vi "Trajectory Builder.vi"() -> ()   [LabVIEW 2025] (continued)
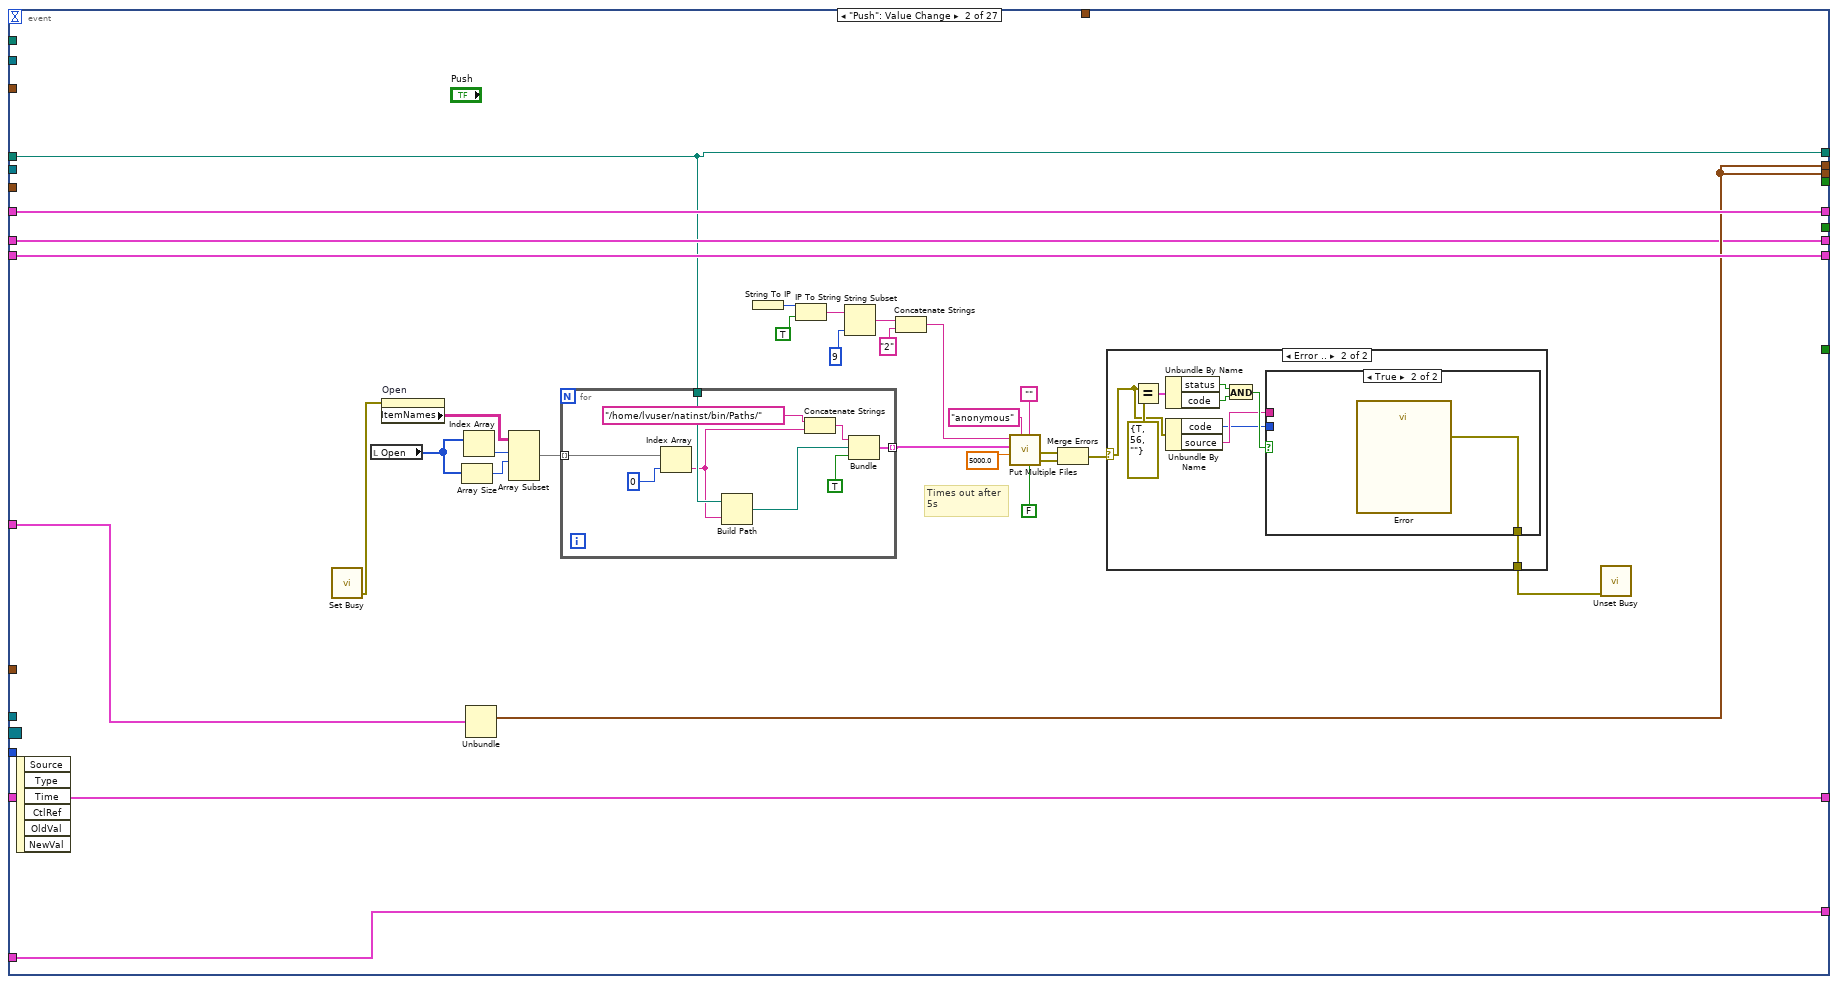
[diagram p4: hidden frame]
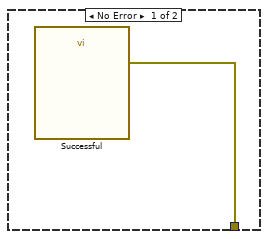
[diagram p5: hidden frame]
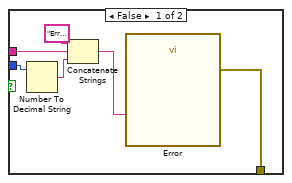
[diagram p6: hidden frame]
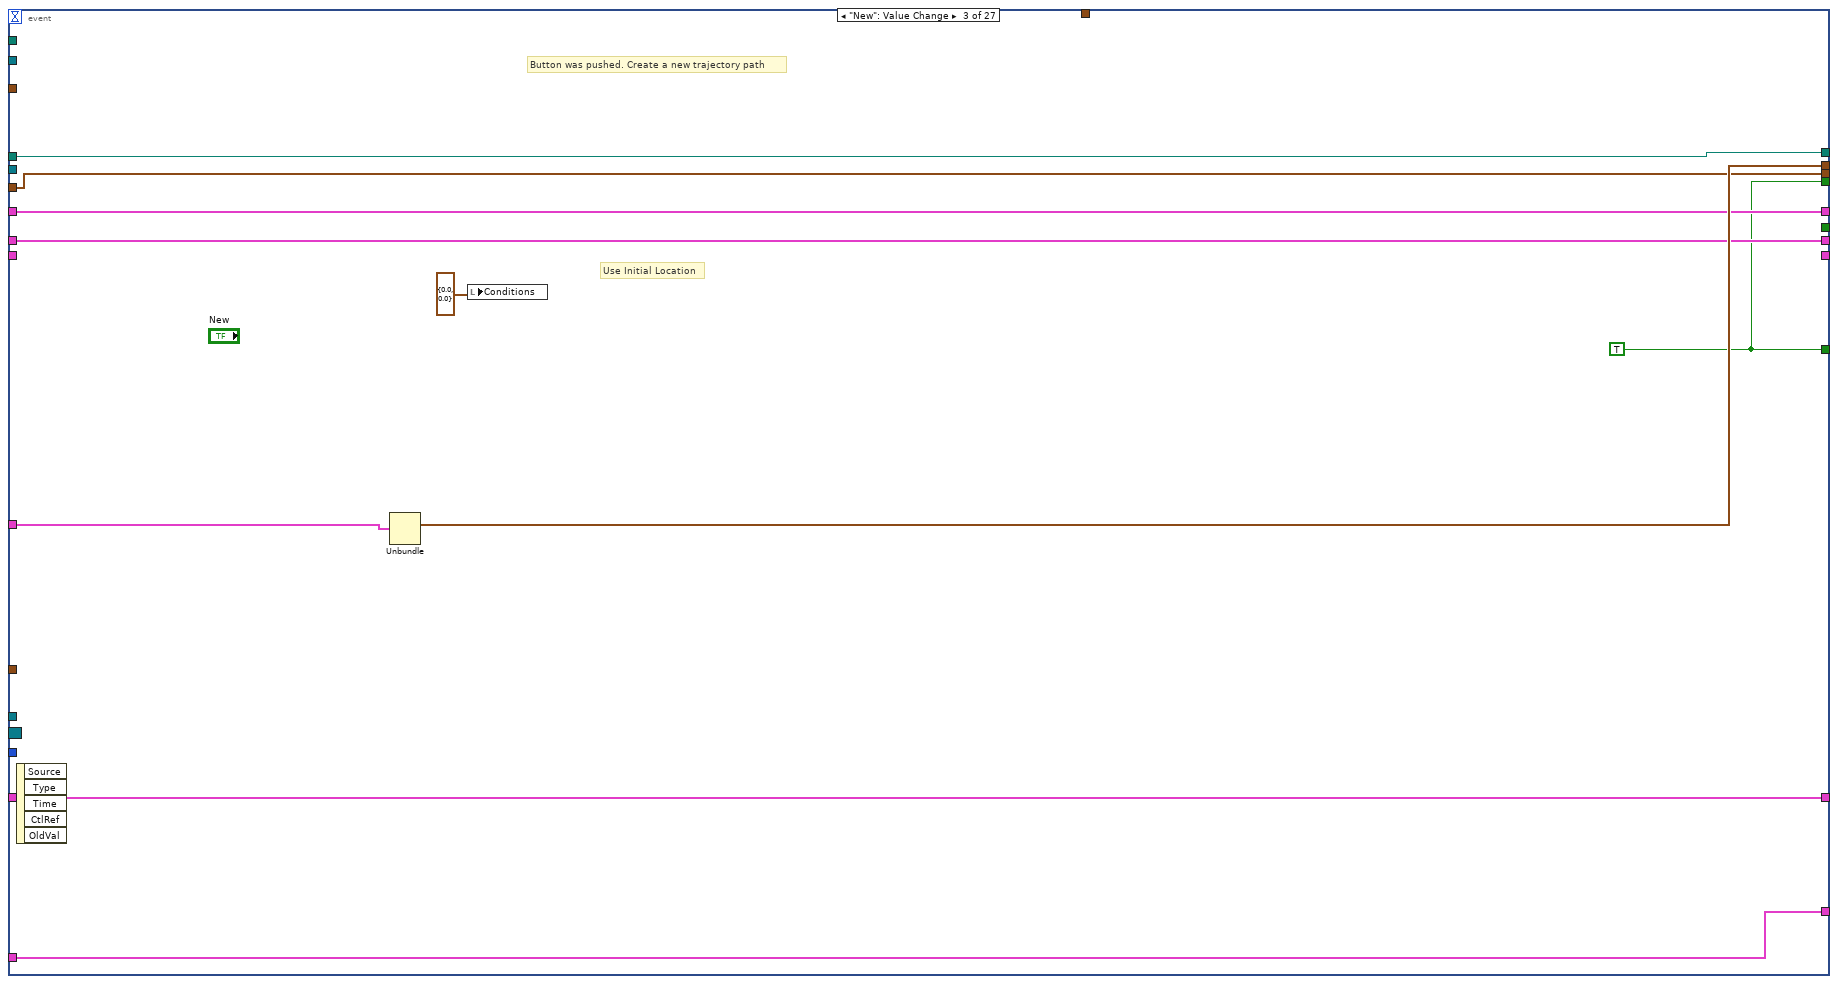
[diagram p7: hidden frame]
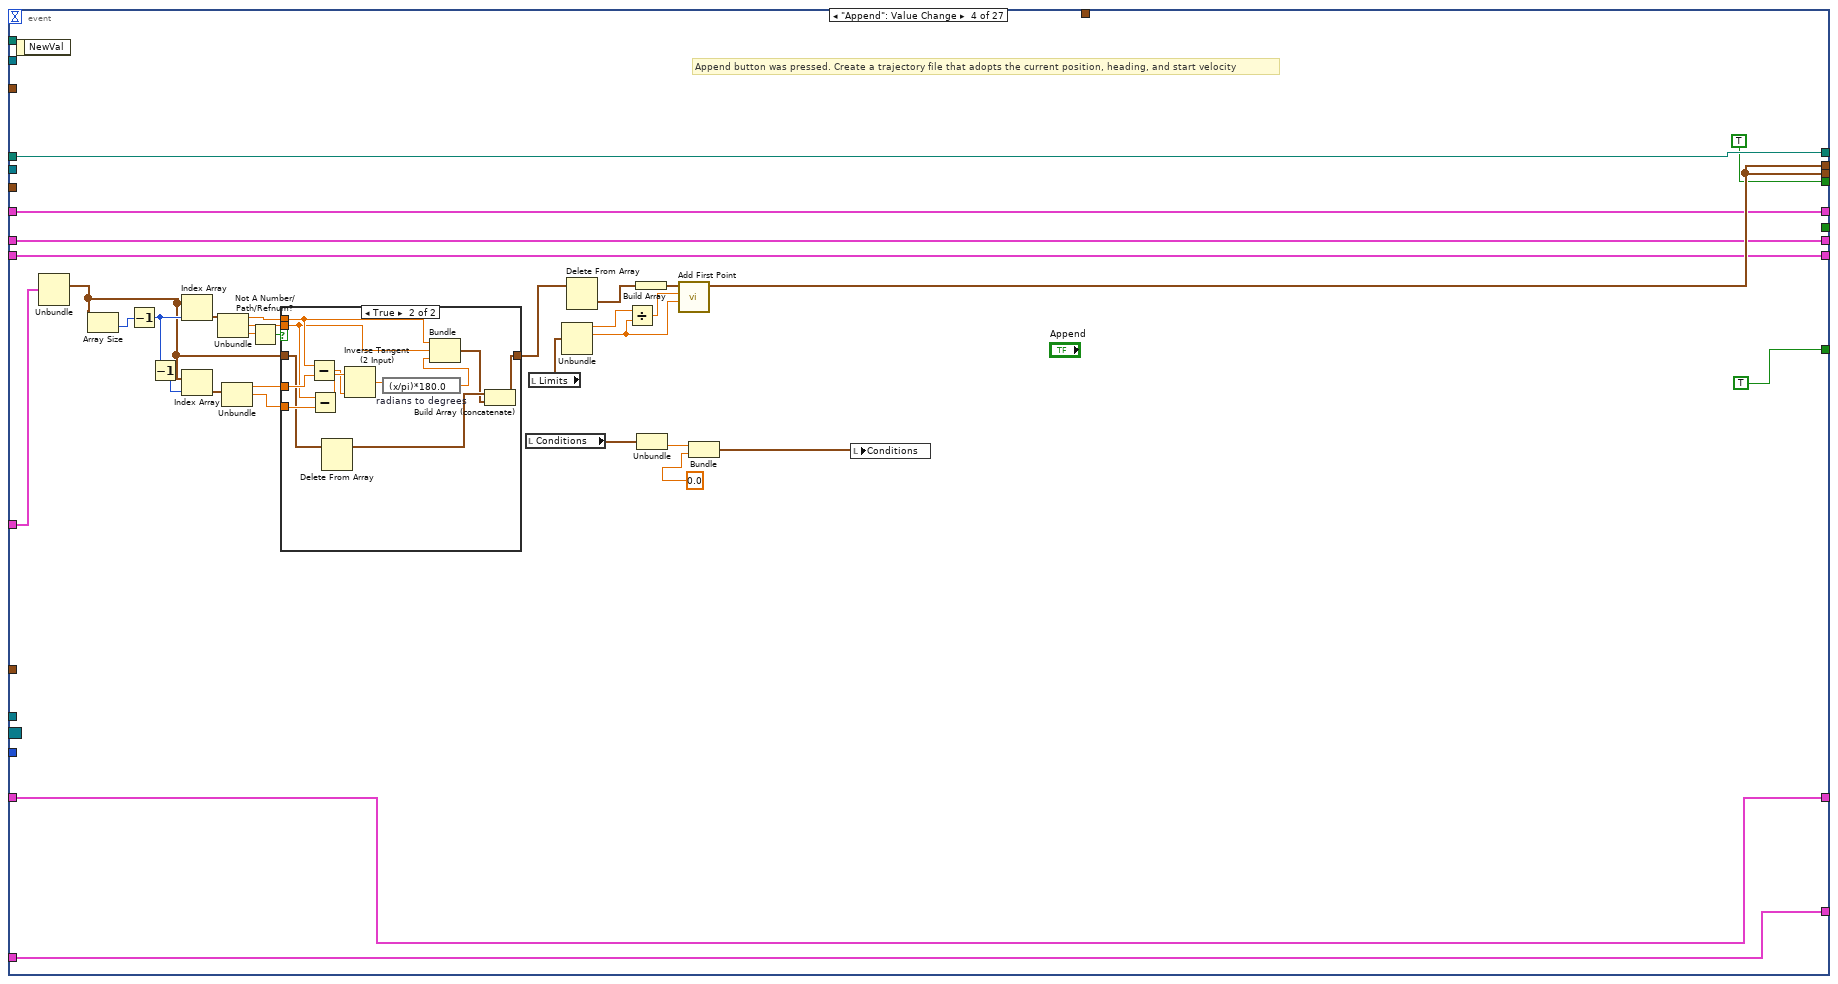
[diagram p8: hidden frame]
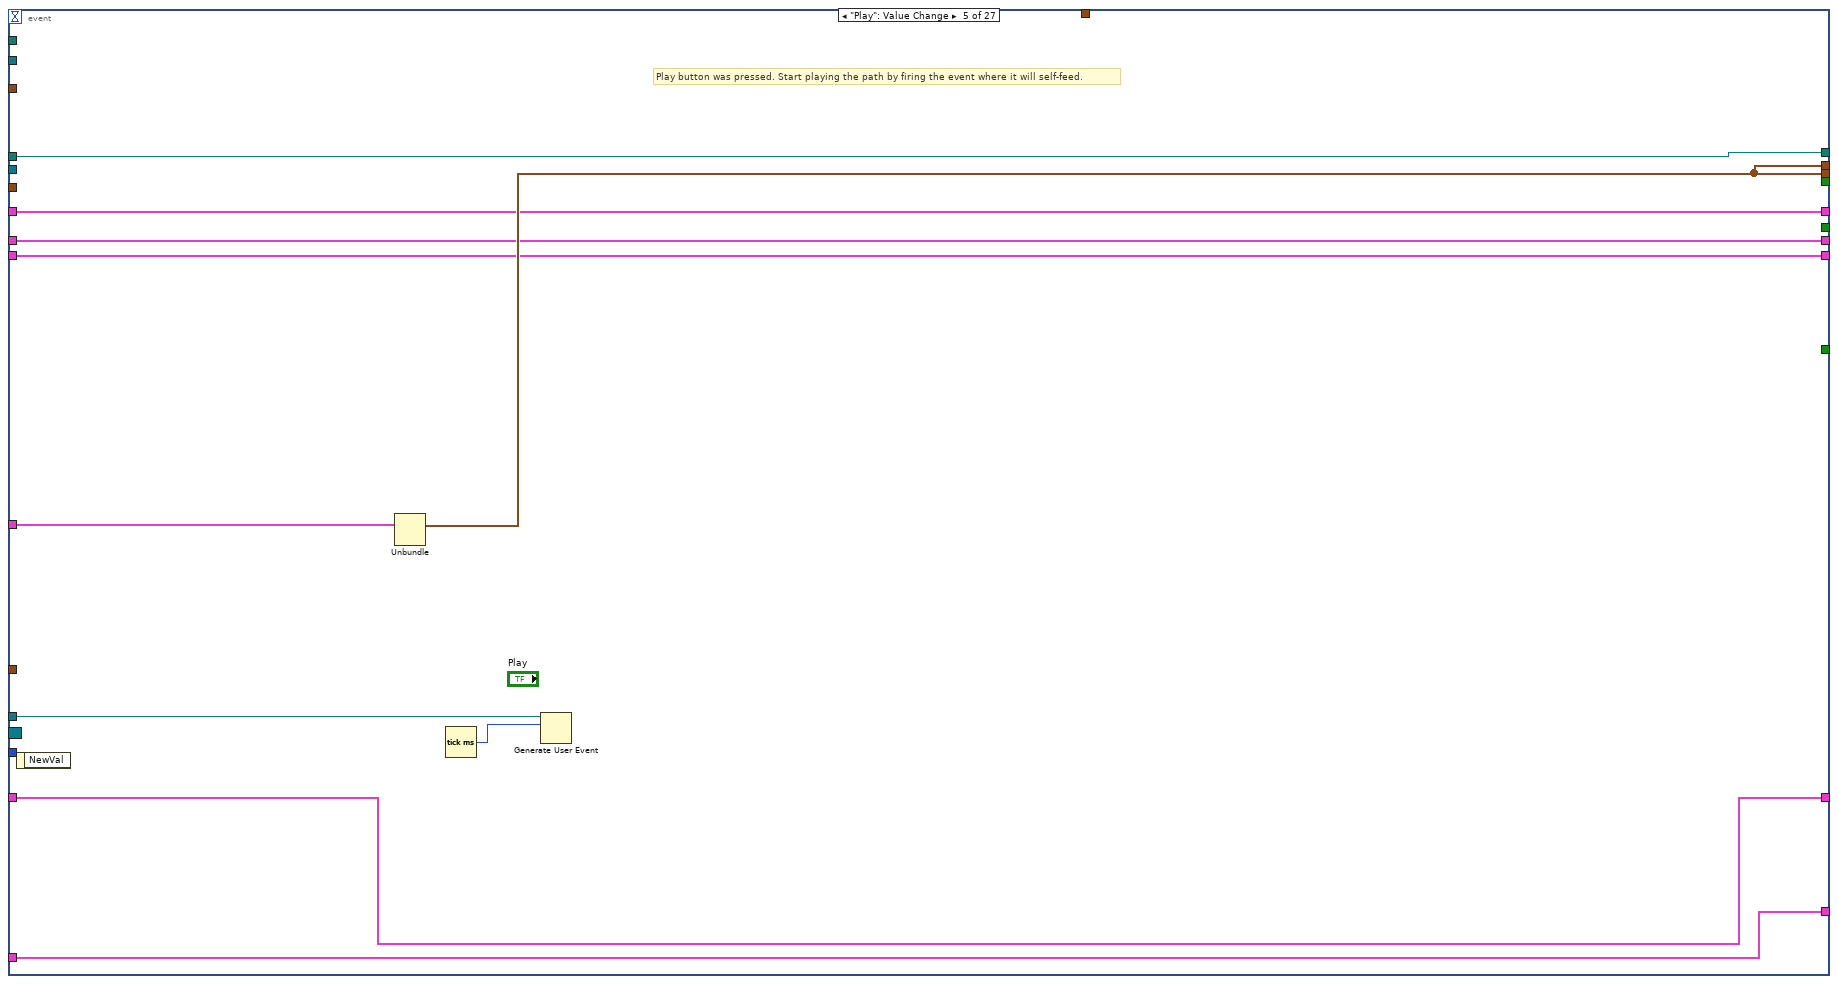
[diagram p10: hidden frame]
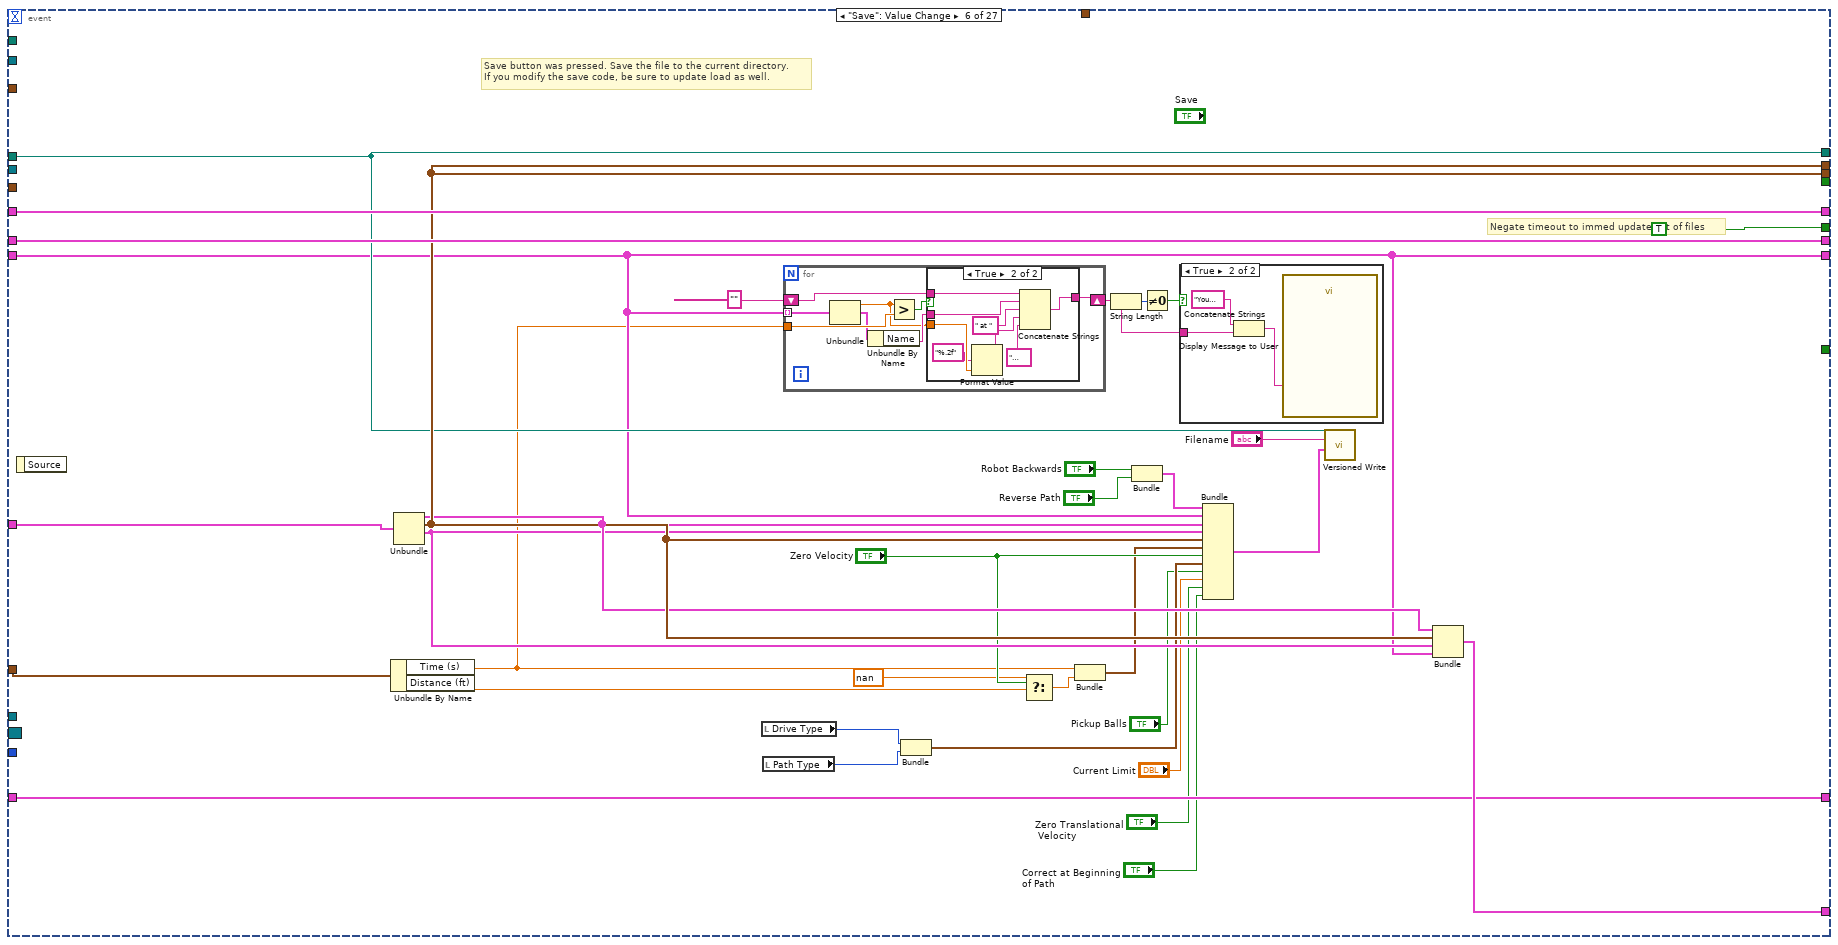
[diagram p11: hidden frame]
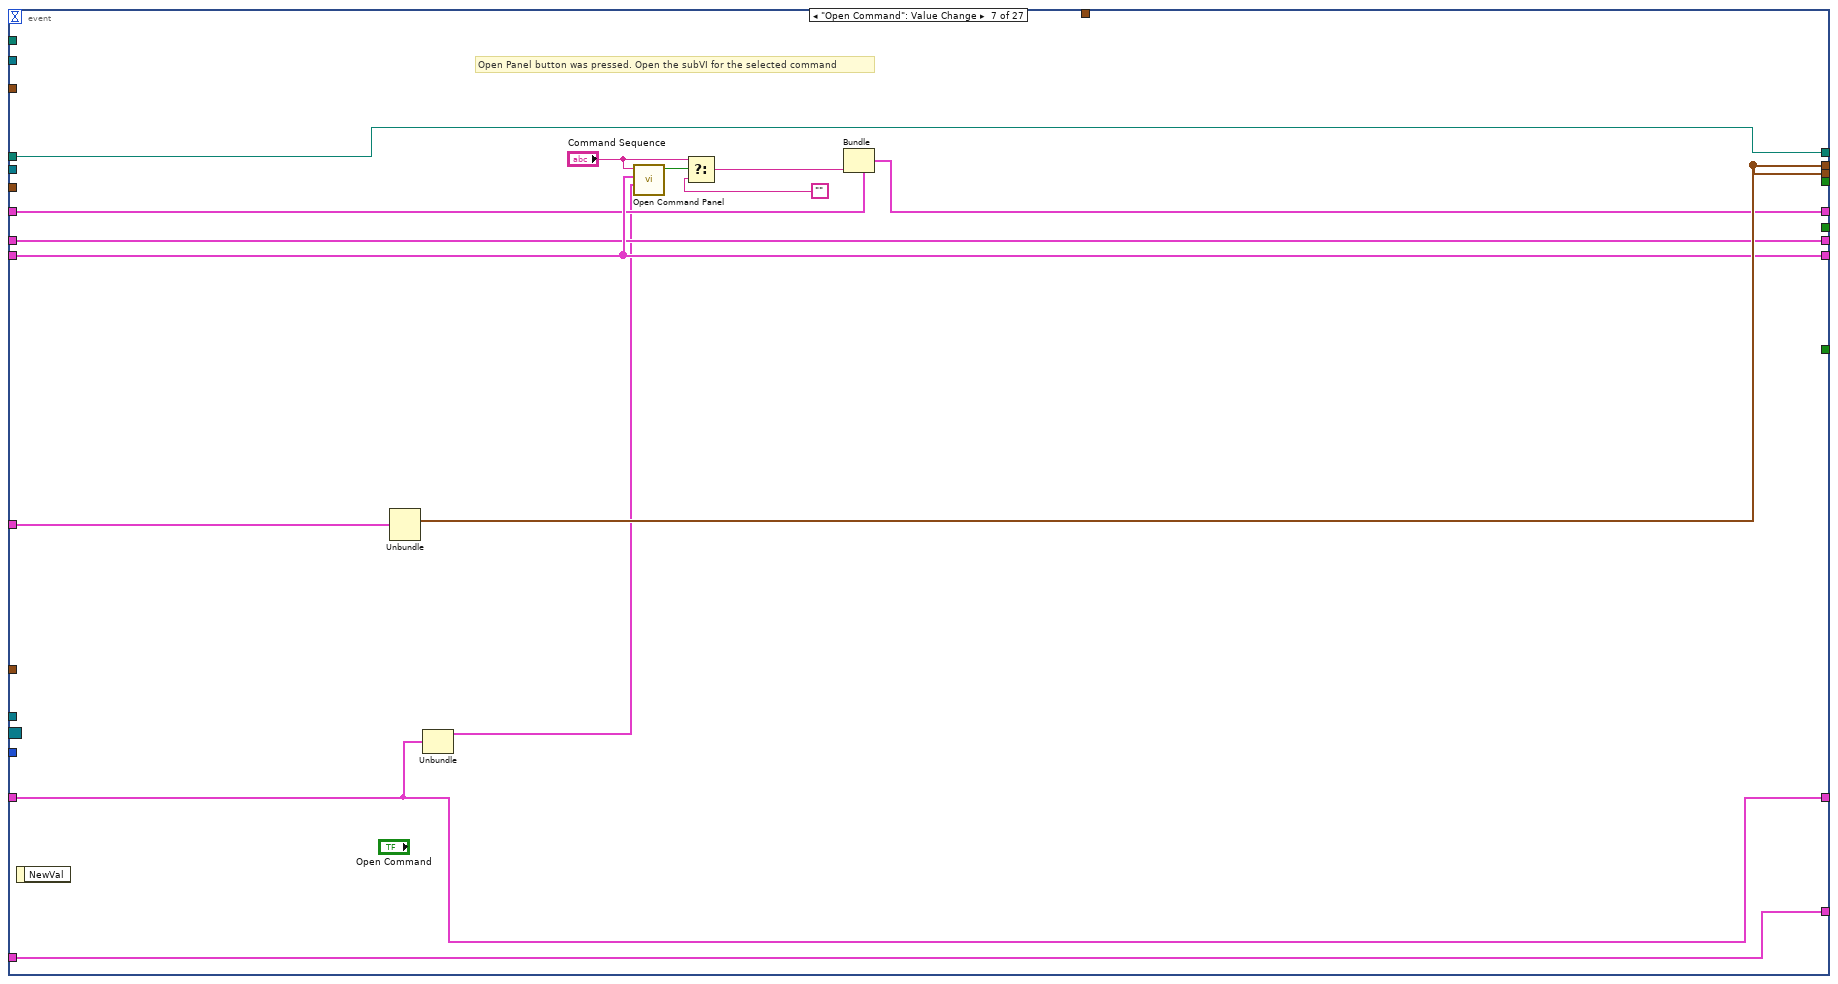
[diagram p14: hidden frame]
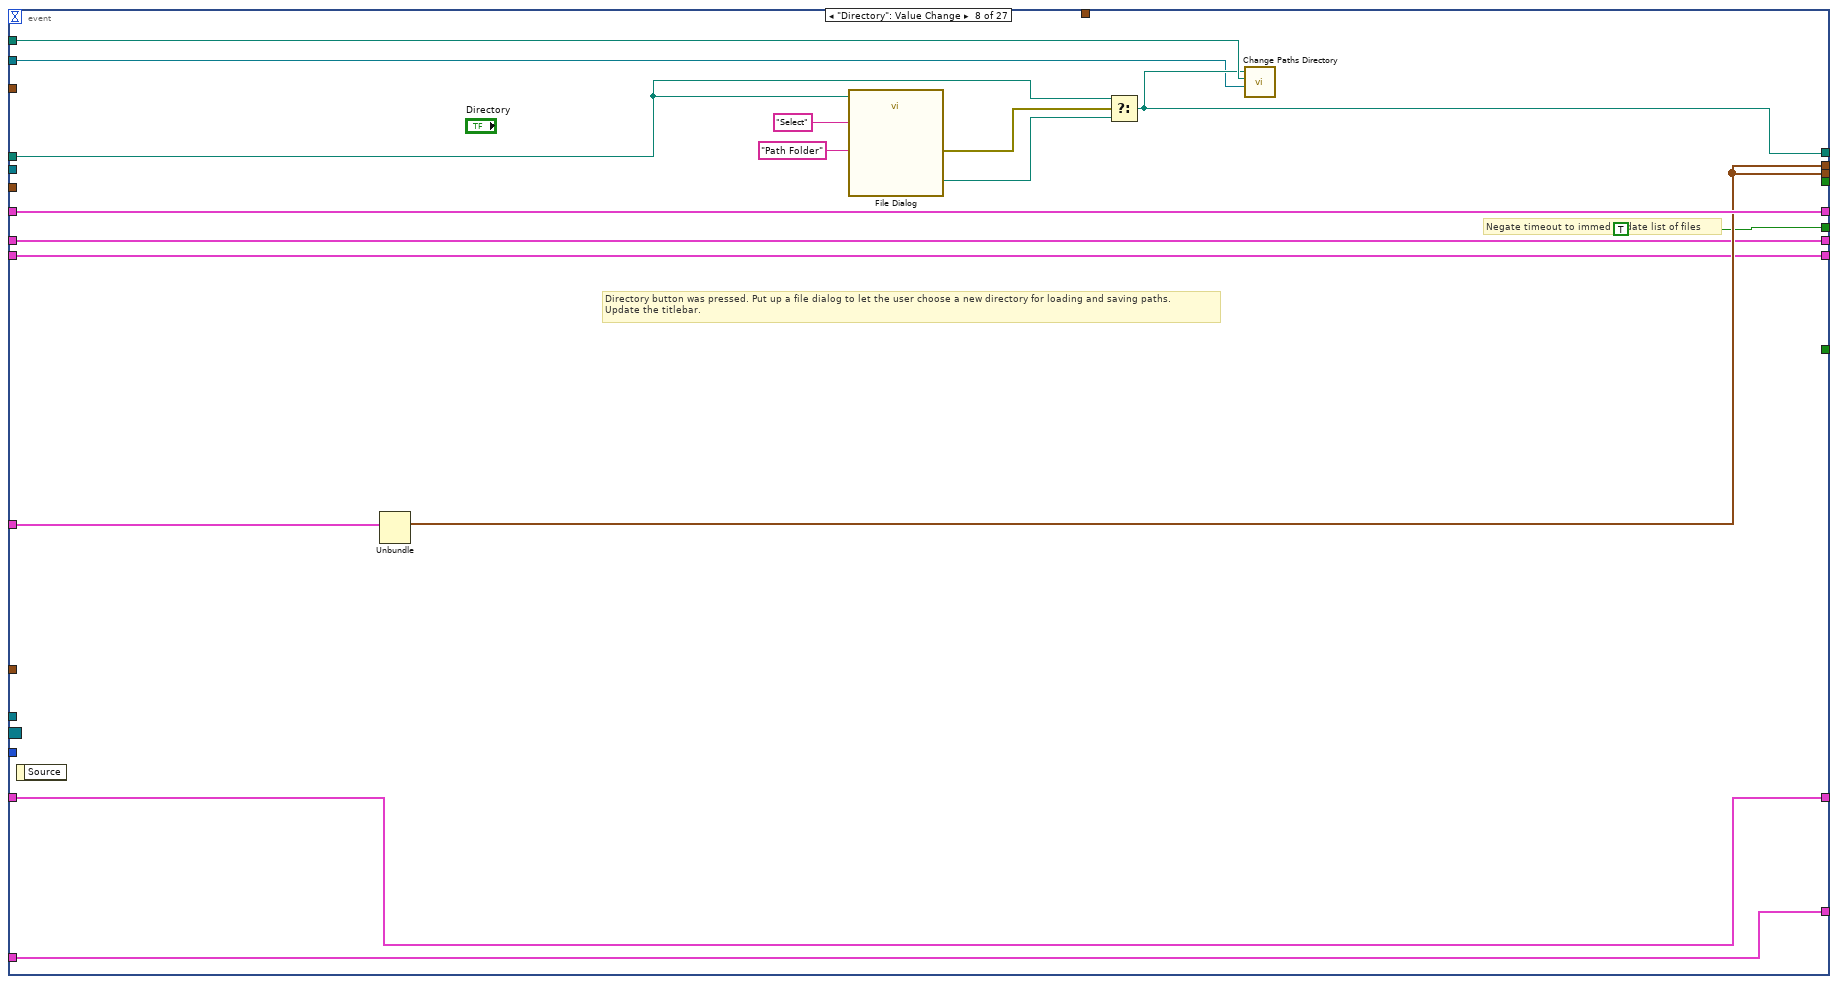
[diagram p15: hidden frame]
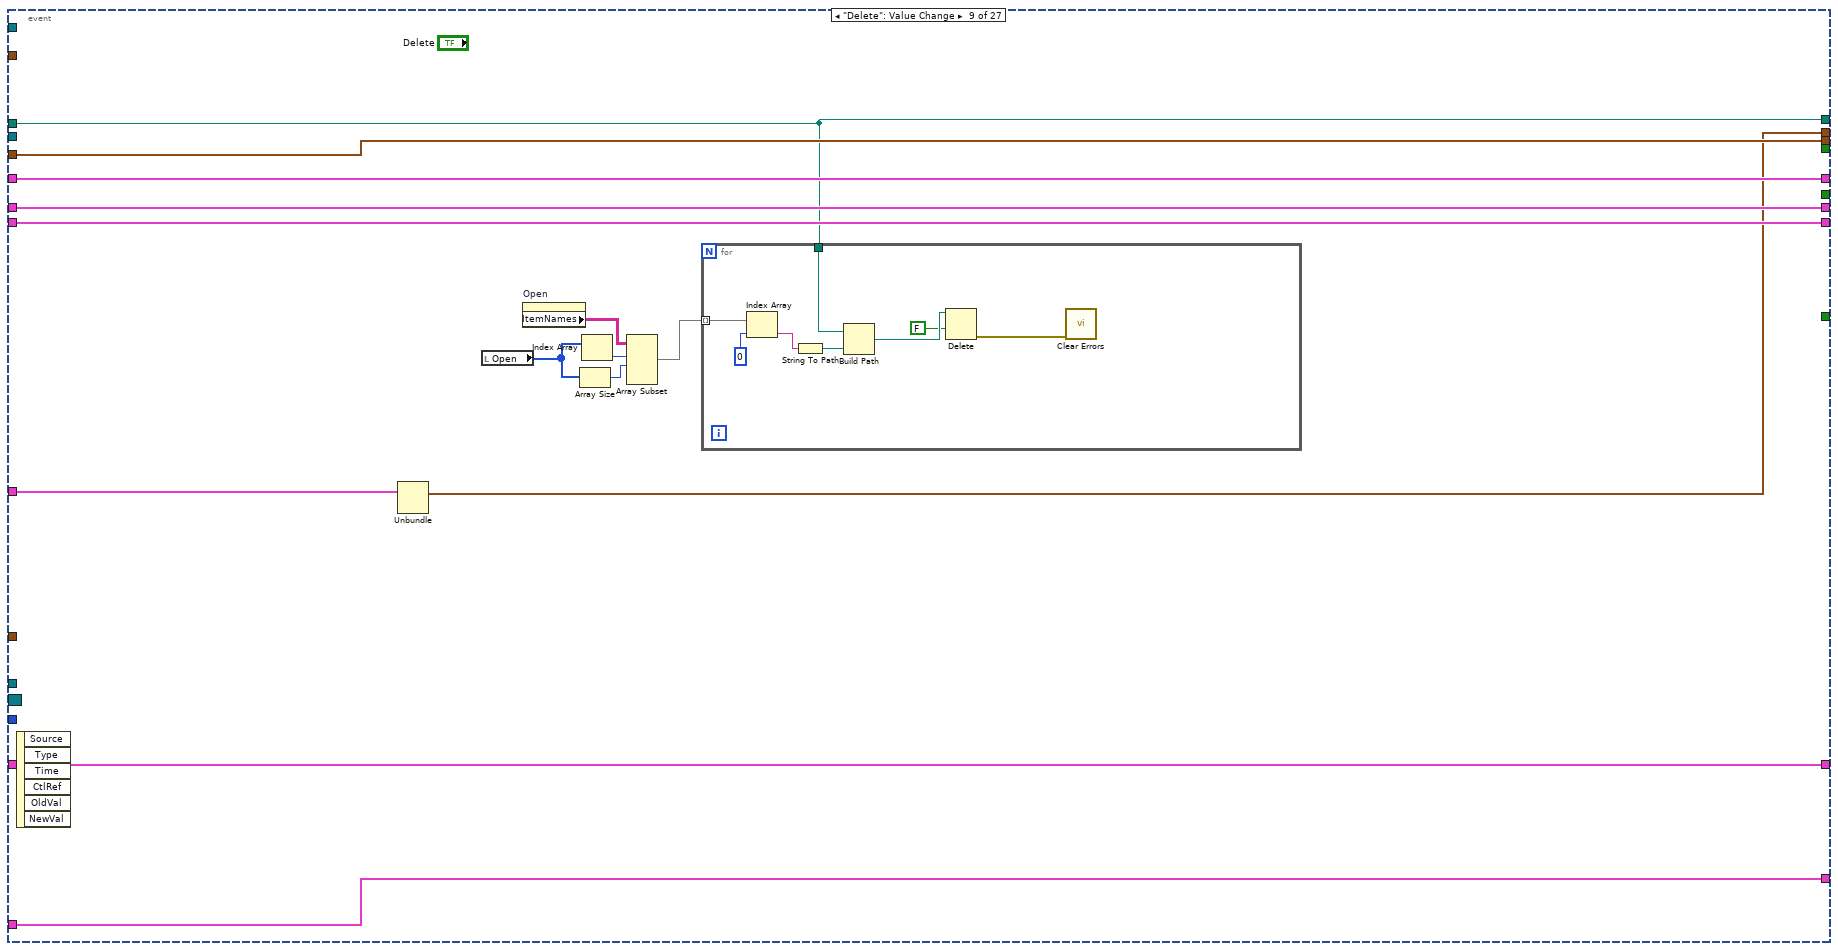
[diagram p16: hidden frame]
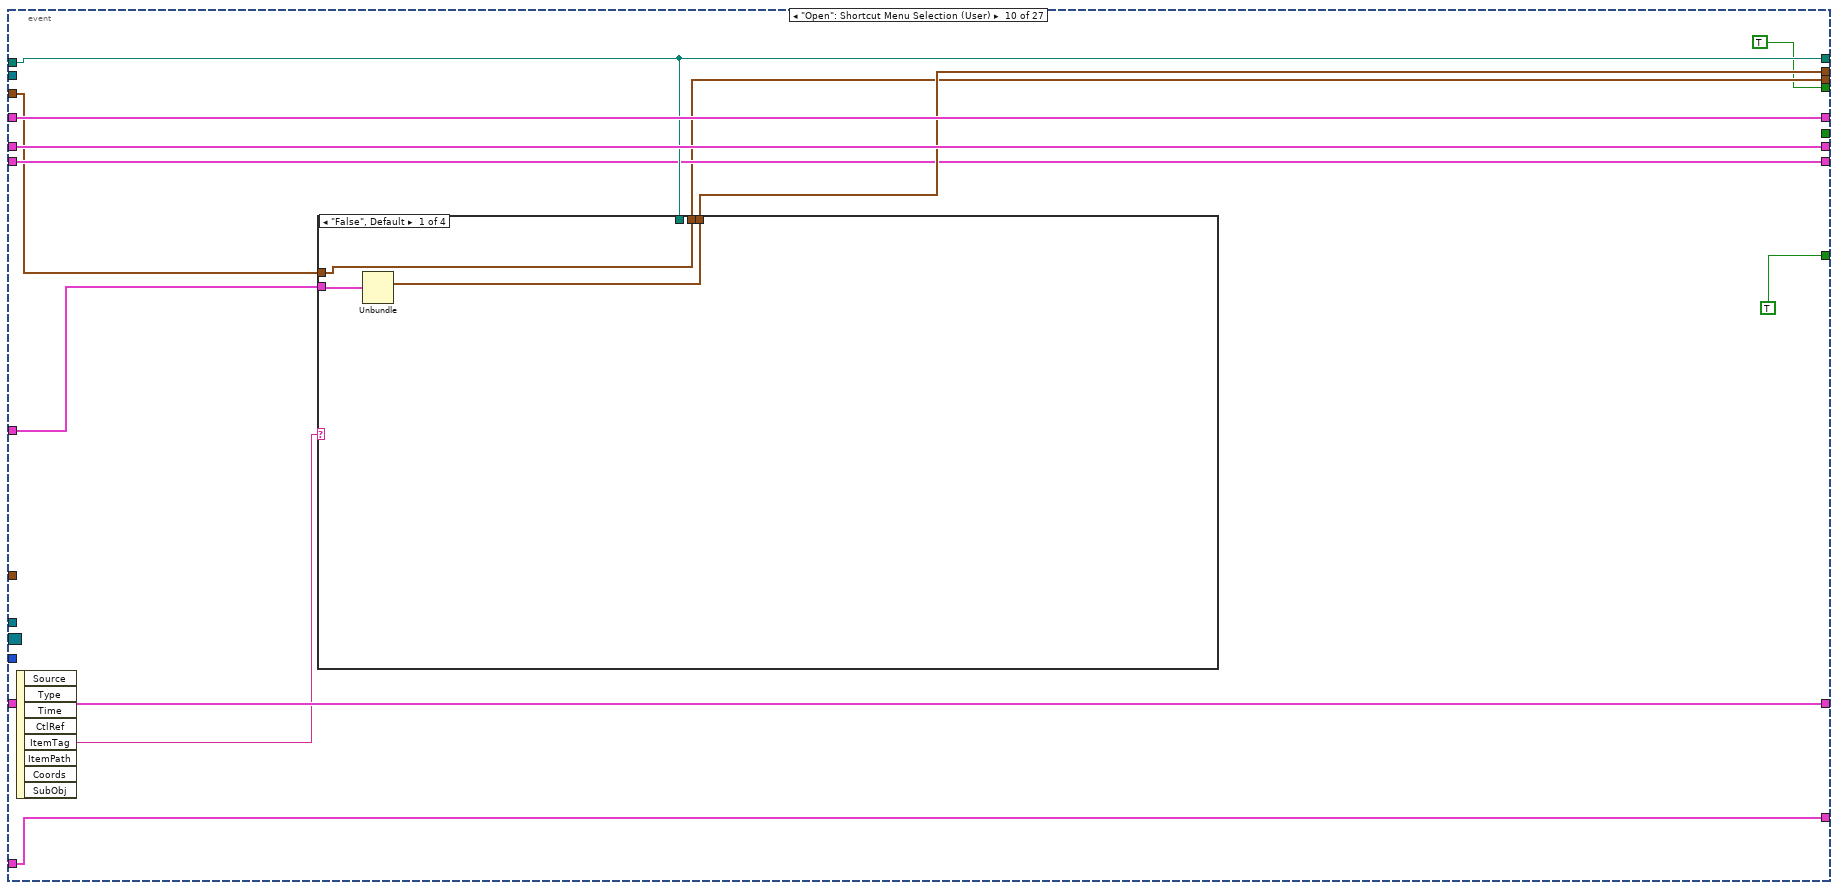
[diagram p17: hidden frame]
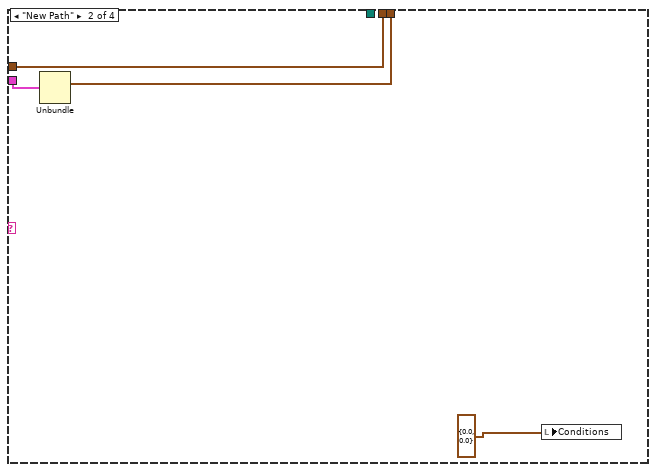
[diagram p18: hidden frame]
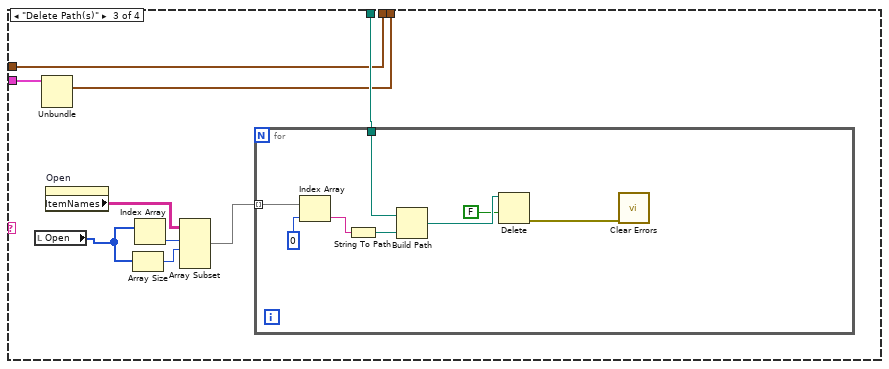
[diagram p19: hidden frame]
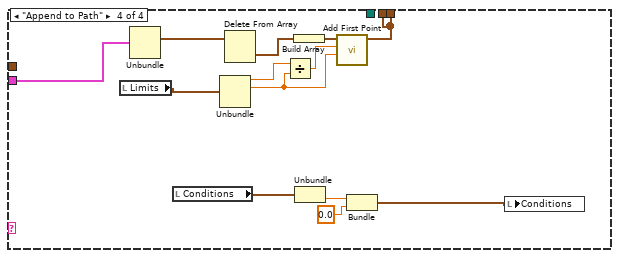
[diagram p20: hidden frame]
    n508 = flat-sequence {
      tunnel: ["Time (s)"] -> w113
      tunnel: ["Sample Period (s)"] -> w86
      tunnel: ["Limits"] -> w65
      tunnel: ["Conditions"] -> w51
      tunnel: [w128] -> w75
      tunnel: ["Overrides"] -> w50
      tunnel: w79 -> [w128]
      tunnel: w78 -> [w130]
      tunnel: ["Hide Path"] -> w69
      tunnel: ["Stoopid Overlap %"] -> w68
      tunnel: ["Angular Limits"] -> w49
      tunnel: [w122] -> w46
      frame #0 {
        n509 = control-ref of="Command Sequence"() -> (w131:refnum<vi>)
        n510 = global write "Global Settings.vi" "> 90?"("Allow Angles > 90") -> ()
        n511 = global write "Global Settings.vi" "Turn Angle Limit (deg)"("Turn Angle Limit (deg)") -> ()
        n512 = call "Format Tree.vi"("Update"=w130, "Commands"=w128, "Tree Refnum"=w131) -> ()  [unwired: 9 in]
        n513 = local read "Overrides"() -> (w122:T8)
      }
    }
    n514 = Unbundle(w65) -> ("Accel (fps^2)"=w64:dbl)  [unwired: 3 out]
    n515 = Divide(x=w113, y=w86) -> (x/y=w106:dbl)
    n516 = Bundle("Sample Period (s)"=w86, "Limits"=w65, "Conditions"=w51, "Overrides"=w50, "Angular Limits"=w49) -> (w66:T14)  [unwired: 1 in]
    n517 = call "Enforce Robot Rules.vi"("max V"=w71, "Drive Type"="Drive Type", "Overrides"=w46, "turn accel"=w64, "Disable"=w59, "New Points"=w108, "Original Points"=w107) -> ("Overrides Out"=w52:T8, "Points out"=w48:cluster{"x":dbl, "y":dbl, "th":dbl}[])  [unwired: 3 in]
    n518 = call "GenNewTraj.vi"("Drive Type"="Drive Type", "Turn Rate"="Turn Rate (Bezier)", "Stoopid Overlap %"=w68, "Path Type"="Path Type", "Parameters"=w66, "Points in"=w48) -> ("Time & Dist"=w58:cluster{"Time (s)":dbl, "Distance (ft)":dbl}, "Valid"=w87:bool, "Trajectory Data"=w95:T12, "Updated Waypoints"=w99:cluster{"x":dbl, "y":dbl, "th":dbl}[])  [unwired: 2 in]
    "Trajectory Data" <- w95
    n519 = local write "WayPoints"(w48) -> ()
    n520 = local write "Overrides"(w52) -> ()
    n521 = Unbundle(w58) -> ("Time (s)"=w56:dbl, "Distance (ft)"=→"Distance (ft)":dbl)
    "Duration (s)" <- w56
    n522 = Unbundle(w93) -> ("Hover Object"=w92:T17)  [unwired: 2 out]
    n523 = Bundle(cluster=T20 {"Trajectory Data"=[], "Updated Waypoints"=[], {"Sample Period (s)"=0.0, "Limits"={"Velocity (fps)"=0.0, "Accel (fps^2)"=0.0, "Jerk (fps^3)"=0.0, "StoopidFast (fps)"=0.0}, "Conditions"={"vInitial (fps)"=0.0, "vFinal (fps)"=0.0}, "Overrides"=[], "Angular Limits"={"Velocity (deg/s)"=6.0, "Accel (deg/s^2)"=15.0, "Jerk (deg/s^3)"=150.0}}, "Commands out"=[]} ("output cluster"), "Trajectory Data"=w95, "Updated Waypoints"=w99, w66, "Commands out"=w75) -> (w53:T20)
    n524 = property on="Time (s)" class="Slide (strict)"("Scale.Minimum"=0.0 ("Scale.Range:Minimum"), "Scale.Maximum"=w56) -> ()  [unwired: 2 in, 2 out]
    n525 = call "Draw Trajectory.vi"("Robot Index"=w106, "Hide Path"=w69, "new picture in"=picture data[5B] ("new picture"), "Trajectory Data"=w95, "Picture in"=w116) -> ("Path Points"=w100:cluster{"x":dbl, "y":dbl}[], "Output Point"=w112:T39, "new picture"=w114:picture)  [unwired: 4 in]
    n526 = call "Draw Shapes.vi"("Path Points"=w100, "Sample Period (s)"=w86, "Output Point"=w112, "Commands"=w75, "Results"=w92, "new picture in"=w114, "Points"=w99, "Picture in"=w116) -> ("new picture out"=→"Picture":picture)  [unwired: 3 in]
    n527 = call "Update Annotations.vi"("Sample Period"=w86, "Commands"=w75, "Trajectory Data"=w95, "Robot Pt Index"=w106) -> ("Redraw"=w77:bool, "Velocity Trace"=w76:dbl[], "Annotation Data"=w105:T40)  [unwired: 5 in]
    n528 = case shown="True" w77 {
      tunnel: w105 -> [_ w1156]
      tunnel: w76 -> [_ w1155]
      frame False {
      }
      frame True {
        n529 = property on="fps" class="WFGraph (strict)"("AnntList"=w1156) -> ()  [unwired: 2 in, 2 out]
        "fps" <- w1155
      }
    }
    n530 = disable-structure shown="Disabled" {
      disable-tunnel: w87 -> [w119 _]
      frame Disabled {
        n531 = Select(t=cluster{u32, u32}[] [{14869218, 14869218}] ("Colors [4]"), s=w119, f=cluster{u32, u32}[] [{6094681, 6094681}] ("Colors [4]")) -> ()  [unwired: 1 out]
      }
      frame Enabled {
      }
    }
    n532 = control-ref of="Save"() -> (w62:refnum<vi>)
    n533 = Select(t=0, s=w88, f=2000) -> (s? t:f=w89:i32)
    n534 = call "Saved Checker.vi"("comp B"=w101, "comp A"=w53, "Save button ref"=w62) -> ()  [unwired: 1 in]
  }
  n535 = local write "Time (s)"(0.0 ("Time")) -> ()
